vi "CRYO_MASTER_FULL_RUN3.vi"() -> ()   [LabVIEW 2017] (continued)
            n626 = Index Array(array=w1254, index=w1253) -> (element=→"TIP7":dbl)
          }
          frame #44 {
            n627 = Search 1D Array(1D array=w1261, element=T14."TTH1" ("SensorLocations")) -> (index of element=w1258:i32)  [unwired: 1 in]
            n628 = Index Array(array=w1259, index=w1258) -> (element=→"TTH1":dbl)
          }
          frame #45 {
            n629 = Search 1D Array(1D array=w1266, element=T14."TTH2" ("SensorLocations")) -> (index of element=w1263:i32)  [unwired: 1 in]
            n630 = Index Array(array=w1264, index=w1263) -> (element=→"TTH2":dbl)
          }
          frame #46 {
            n631 = Search 1D Array(1D array=w1271, element=T14."TTH3" ("SensorLocations")) -> (index of element=w1268:i32)  [unwired: 1 in]
            n632 = Index Array(array=w1269, index=w1268) -> (element=→"TTH3":dbl)
          }
          frame #47 {
            n633 = Search 1D Array(1D array=w1276, element=T14."TTH4" ("SensorLocations")) -> (index of element=w1273:i32)  [unwired: 1 in]
            n634 = Index Array(array=w1274, index=w1273) -> (element=→"TTH4":dbl)
          }
          frame #48 {
            n635 = Search 1D Array(1D array=w1281, element="SensorLocation 1") -> (index of element=w1278:i32)  [unwired: 1 in]
            n636 = Index Array(array=w1279, index=w1278) -> (element=→"Temperature 1":dbl)
          }
          frame #49 {
            n637 = Search 1D Array(1D array=w1286, element="SensorLocation 2") -> (index of element=w1283:i32)  [unwired: 1 in]
            n638 = Index Array(array=w1284, index=w1283) -> (element=→"Temperature 2":dbl)
          }
        }
      }
      frame #1 {
        n639 = stacked-sequence {
          tunnel: w1288 -> [w1293 w1298 w1303 w1308 w1313 w1318 w1323 w1328 w1333 w1338 w1343 w1348 w1353 w1358 w1363 w1368 w1373 w1378 w1383]
          tunnel: w1287 -> [w1290 w1296 w1302 w1307 w1312 w1316 w1321 w1326 w1331 w1336 w1341 w1346 w1350 w1355 w1360 w1365 w1370 w1375 _]
          tunnel: w1287 -> [_ _ _ _ _ _ _ _ _ _ _ _ _ _ _ _ _ _ w1381]
          frame #0 {
            n640 = Search 1D Array(1D array=w1293, element="Insulation vacuum") -> (index of element=w1291:i32)  [unwired: 1 in]
            n641 = Index Array(array=w1290, index=w1291) -> (element=→"P_ins" →"P (insulation)":dbl)
          }
          frame #1 {
            n642 = Search 1D Array(1D array=w1298, element="4K reservoir pressure") -> (index of element=w1295:i32)  [unwired: 1 in]
            n643 = Index Array(array=w1296, index=w1295) -> (element=→"P_4Kres" →"P (4K reservoir)":dbl)
          }
          frame #2 {
            n644 = Search 1D Array(1D array=w1303, element="3He inlet pressure") -> (index of element=w1301:i32)  [unwired: 1 in]
            n645 = Index Array(array=w1302, index=w1301) -> (element=→"P_3HeIN" →"P (3He IN)":dbl)
          }
          frame #3 {
            n646 = Search 1D Array(1D array=w1308, element="Shield return press.") -> (index of element=w1306:i32)  [unwired: 1 in]
            n647 = Index Array(array=w1307, index=w1306) -> (element=→"P_SldRTN" →"P (shield return)":dbl)
          }
          frame #4 {
            n648 = Search 1D Array(1D array=w1313, element="3He pot pressure") -> (index of element=w1311:i32)  [unwired: 1 in]
            n649 = Index Array(array=w1312, index=w1311) -> (element=→"P_3Hepot" →"P (3He pot)":dbl)
          }
          frame #5 {
            n650 = Search 1D Array(1D array=w1318, element="1Kpot pressure") -> (index of element=w1315:i32)  [unwired: 1 in]
            n651 = Index Array(array=w1316, index=w1315) -> (element=→"P_1Kpot" →"P (1K pot)":dbl)
          }
          frame #6 {
            n652 = Search 1D Array(1D array=w1323, element="Dewar pressure") -> (index of element=w1320:i32)  [unwired: 1 in]
            n653 = Index Array(array=w1321, index=w1320) -> (element=→"P_Dewar" →"P (Dewar)":dbl)
          }
          frame #7 {
            n654 = Search 1D Array(1D array=w1328, element="HEX7 out pressure") -> (index of element=w1325:i32)  [unwired: 1 in]
            n655 = Index Array(array=w1326, index=w1325) -> (element=→"P_HEX7OUT" →"P (HEX7 out)":dbl)
          }
          frame #8 {
            n656 = Search 1D Array(1D array=w1333, element="Diff pressure HEX4") -> (index of element=w1330:i32)  [unwired: 1 in]
            n657 = Index Array(array=w1331, index=w1330) -> (element=→"DP_HEX4" →"DP HEX4":dbl)
          }
          frame #9 {
            n658 = Search 1D Array(1D array=w1338, element="Diff pressure HEX5") -> (index of element=w1335:i32)  [unwired: 1 in]
            n659 = Index Array(array=w1336, index=w1335) -> (element=→"DP_HEX5" →"DP HEX5":dbl)
          }
          frame #10 {
            n660 = Search 1D Array(1D array=w1343, element="3He pump exhaust flow") -> (index of element=w1340:i32)  [unwired: 1 in]
            n661 = Index Array(array=w1341, index=w1340) -> (element=→"F_1" →"F1 (3He pump exhaust) flow":dbl)
          }
          frame #11 {
            n662 = Search 1D Array(1D array=w1348, element="Shield flow") -> (index of element=w1345:i32)  [unwired: 1 in]
            n663 = Index Array(array=w1346, index=w1345) -> (element=→"F_2" →"F2 (shield flow)":dbl)
          }
          frame #12 {
            n664 = Search 1D Array(1D array=w1353, element="4He return flow from HEX7") -> (index of element=w1351:i32)  [unwired: 1 in]
            n665 = Index Array(array=w1350, index=w1351) -> (element=→"F_3" →"F3 (4He rtn flw via HEX7)":dbl)
          }
          frame #13 {
            n666 = Search 1D Array(1D array=w1358, element="3He incoming flow into HEX7") -> (index of element=w1356:i32)  [unwired: 1 in]
            n667 = Index Array(array=w1355, index=w1356) -> (element=→"F_4" →"F4 (3He in to HEX7)":dbl)
          }
          frame #14 {
            n668 = Search 1D Array(1D array=w1363, element="1Kpot pump exhaust flow") -> (index of element=w1361:i32)  [unwired: 1 in]
            n669 = Index Array(array=w1360, index=w1361) -> (element=→"F_5" →"F5 (1K pump ex.)":dbl)
          }
          frame #15 {
            n670 = Search 1D Array(1D array=w1368, element="4K reservoir level") -> (index of element=w1366:i32)  [unwired: 1 in]
            n671 = Index Array(array=w1365, index=w1366) -> (element=→"L3" →"He level (4K)":dbl)
          }
          frame #16 {
            n672 = Search 1D Array(1D array=w1373, element="1K pot level") -> (index of element=w1371:i32)  [unwired: 1 in]
            n673 = Index Array(array=w1370, index=w1371) -> (element=→"L(1K) (a1)" →"He level (1K)":dbl)
          }
          frame #17 {
            n674 = Search 1D Array(1D array=w1378, element="1K pot (b)") -> (index of element=w1376:i32)  [unwired: 1 in]
            n675 = Index Array(array=w1375, index=w1376) -> (element=→"1K pot(b1)" →"He level (1K) b":dbl)
          }
          frame #18 {
            n676 = case shown="False" TRUE {
              tunnel: w1383 -> [w1388 _]
              tunnel: "3He pot" -> [w1387 w1392]
              tunnel: w1381 -> [w1385 _]
              tunnel: [w1384 w1391] -> w1380
              frame False {
                n677 = Search 1D Array(1D array=w1388, element=w1387) -> (index of element=w1386:i32)  [unwired: 1 in]
                n678 = Index Array(array=w1385, index=w1386) -> (element=w1384:dbl)
              }
              frame True {
                n679 = local read "Labels (HP34401 LM)"() -> (w1393:string[])
                n680 = local read "LastData (HP34401 LM)"() -> (w1389:dbl[])
                n681 = Search 1D Array(1D array=w1393, element=w1392) -> (index of element=w1390:i32)  [unwired: 1 in]
                n682 = Index Array(array=w1389, index=w1390) -> (element=w1391:dbl)
              }
            }
            "3He pot level" <- w1380
            "He level (3He)" <- w1380
          }
        }
      }
    }
    n683 = case shown="True" w848 {
      tunnel: [w1954 w1966] -> w908
      tunnel: [w1944 w1965] -> w916
      tunnel: [w1953 w1964] -> w909
      tunnel: [w1952 timestamp[] [] ("TimeArray")] -> w878
      tunnel: [w1951 dbl[][] [] ("DataArray")] -> w876
      tunnel: w918 -> [w1950 w1961]
      tunnel: w917 -> [w1949 w1960]
      tunnel: w842 -> [w1945 _]
      tunnel: w845 -> [_ w1955]
      frame False {
        n684 = local read "Record interval"() -> (w1942:i64)
        n685 = call-dynamic "LSI336Data_measure.vi"("LSI336Data in"=w1950, "MeasurementIndex"=w1945, "error in (no error)"=w1949, "save every ... measurements"=w1942) -> ("Active?"=→"Active?\n(LSI336)":bool[], "TimeMeasuremeent"=→"Time of Last Measurement (LSI336)":timestamp, "LSI336Data out"=w1953:refnum<class "LSI336Data.lvclass">, "LastData"=→"Last Data \nLSI336":dbl[], "LastMeasurementConfig"=→"LastMeasurementConfig (336)":T17, "DataArray"=w1951:dbl[][], "Status"=w1944:u16, "TimeArray"=w1952:timestamp[], "error out"=w1954:errorcluster)  [unwired: 3 in]
      }
      frame True {
        n686 = local read "RUN Identifier"() -> (w1956:string)
        n687 = call-dynamic "LSI336Data_initialize.vi"("LSI336Data in"=w1961, "RunIdentifier"=w1956, "InstName"="InstName (LSI336)", "FileFormat"="FileFormat (336)", "LSI336Settings(X, Y)"="LSI336Settings(X,Y)", "error in (no error)"=w1960, "base path"=w1955) -> ("LSI336Data out"=w1964:refnum<class "LSI336Data.lvclass">, "Status"=w1965:T7, "AllLabels"=→"Labels LSI336":string[], "error out"=w1966:errorcluster)  [unwired: 5 in]
      }
    }
    "LSI336 Status" <- w916
    "error out (LSI336)" <- w908
    "TimeArray (LSI336)" <- w878
    "DataArray (336)" <- w876
    n688 = local read "Labels (HP34401 LM) 2"() -> (w841:string[])
    n689 = case shown="False" w848 {
      tunnel: [w2059 w2074] -> w921
      tunnel: [w2054 w2073] -> w938
      tunnel: [w2057 w2072] -> w922
      tunnel: w842 -> [w2058 _]
      tunnel: w937 -> [w2048 w2067]
      tunnel: w936 -> [w2049 w2066]
      tunnel: w845 -> [_ w2065]
      tunnel: [w2046 timestamp[] [] ("TimeArray")] -> w935
      tunnel: [w2045 dbl[][] [] ("DataArray")] -> w934
      frame False {
        w2052 = 24 ("index")
        n690 = local read "Record interval"() -> (w2043:i64)
        n691 = call-dynamic "LSI218Data_measure.vi"("LSI218Data in"=w2049, "MeasurementIndex"=w2058, "error in (no error)"=w2048, "save every ... measurements"=w2043) -> ("TimeMeasuremeent"=→"Time of Last Measurement (LSI218)":timestamp, "Active?"=w2053:bool[], "LSI218Data out"=w2057:refnum<class "LSI218Data.lvclass">, "LastMeasurementConfig"=→"LastMeasurementConfig (218)":T17, "LastData"=w2047:dbl[], "Status"=w2054:u16, "TimeArray"=w2046:timestamp[], "DataArray"=w2045:dbl[][], "error out"=w2059:errorcluster)  [unwired: 3 in]
        "LastData (LSI218)" <- w2047
        n692 = Split 1D Array(array=w2053, index=w2052) -> (first subarray=→"Active?\n (1)":bool[], second subarray=→"Active?\n(2)":bool[])
        n693 = Split 1D Array(array=w2047, index=w2052) -> (first subarray=→"Last Data \nLSI218 (1)":dbl[], second subarray=→"Last Data \nLSI218 (2)":dbl[])
      }
      frame True {
        n694 = local read "RUN Identifier"() -> (w2061:string)
        n695 = call-dynamic "LSI218Data_initialize.vi"("LSI218Settings(A-F)"="LSI218Settings(A-F)", "FileFormat"="FileFormat (218)", "base path"=w2065, "error in (no error)"=w2067, "InstName"="InstName (LSI218)", "RunIdentifier"=w2061, "LSI218Data in"=w2066) -> ("error out"=w2074:errorcluster, "Status"=w2073:T7, "AllLabels"=w2064:string[], "LSI218Data out"=w2072:refnum<class "LSI218Data.lvclass">)  [unwired: 1 in]
        n696 = Split 1D Array(array=w2064, index=24) -> (first subarray=→"Labels LSI218 (1)":string[], second subarray=→"Labels LSI218 (2)":string[])
      }
    }
    "LSI218 Status" <- w938
    "error out (LSI218)" <- w921
    n697 = case shown="True" w848 {
      tunnel: w847 -> [w1010 w1024]
      tunnel: [w1007 w1023] -> w846
      tunnel: w845 -> [_ w1021]
      tunnel: w844 -> [w1009 w1020]
      tunnel: [w1006 w1017] -> w843
      tunnel: w842 -> [w1008 _]
      tunnel: [w1004 dbl[][] [] ("LastDataArray")] -> w839
      tunnel: [w1003 timestamp[] [] ("LastTimeArray")] -> w837
      frame False {
        n698 = call-dynamic "LMData_measure.vi"("error in (no error)"=w1009, "MeasurementInterval(>0)"="LM measurement interval (>0)", "MeasurementIndex"=w1008, "LMData in"=w1010) -> ("error out"=w1006:errorcluster, "LastDataArray"=w1004:dbl[][], "LastMeasurement"=→"LastData (HP34401 LM)":dbl[], "LMData out"=w1007:refnum<class "LMData.lvclass">, "LastTimeArray"=w1003:timestamp[])  [unwired: 3 in]
      }
      frame True {
        n699 = local read "RUN Identifier"() -> (w1022:string)
        n700 = call-dynamic "LMData_initialize.vi"("LMData in"=w1024, "VISA resource name"="VISA (HP34401 LM)", "Labels"="Labels (HP34401 LM)", "FileFormat"="FileFormat (HP34401 LM)", "RunIdentifier"=w1022, "InstName"="InstName (HP34401 LM)", "base path"=w1021, "error in (no error)"=w1020, "LevelCalibration (R0, R1, L0, L1)"="LevelCalibration (R0, R1, L0, L1)", "Active?"="Active? (HP34401 LM)") -> ("LMData out"=w1023:refnum<class "LMData.lvclass">, "error out"=w1017:errorcluster)  [unwired: 4 in]
        "Labels (HP34401 LM) 2" <- "Labels (HP34401 LM)"
      }
    }
    "error out (HP34401 LM)" <- w843
    n701 = Array Size(array=w841) -> (size(s)=w840:i32)
    n702 = for {
      N: w840 -> [_]
      tunnel: w839 -> [w964]
      shift-right: [w951] -> w833
      shift-left: w838 -> [w950]
      shift-right: [w954] -> w835
      shift-left: w838 -> [w955]
      shift-right: [w958] -> w836
      shift-left: w838 -> [w959]
      shift-right: [w953] -> w834
      shift-left: w838 -> [w952]
      tunnel: w837 -> [w962]
      i -> [w963]
      n703 = local read "Plot selecter (HP34401A)\n    1      2     3     4"() -> (w969:bool[][])
      n704 = Index Array(array=w964, index (col)=w963) -> (element=w961:dbl[])  [unwired: 1 in]
      n705 = Bundle("LastTimeArray"=w962, "LastDataArray"=w961) -> (w960:T29)  [unwired: 1 in]
      n706 = Index Array(array=w969, index (row) #1=w963, index (col) #1=0 ("disabled index (col)"), index (row) #2=w963, index (col) #2=1 ("index (col)"), index (row) #3=w963, index (col) #3=2 ("index (col)"), index (row) #4=w963, index (col) #4=3 ("disabled index (col)")) -> (element #1=w957:bool, element #2=w956:bool, element #3=w949:bool, element #4=w948:bool)
      n707 = stacked-sequence {
        tunnel: w960 -> [w971 w978 w989 w997]
        tunnel: w959 -> [w973 _ _ _]
        tunnel: [w972 _ _ _] -> w958
        tunnel: w957 -> [w970 _ _ _]
        tunnel: w956 -> [_ w981 _ _]
        tunnel: w955 -> [_ w980 _ _]
        tunnel: [_ w979 _ _] -> w954
        tunnel: [_ _ w988 _] -> w953
        tunnel: w952 -> [_ _ w987 _]
        tunnel: [_ _ _ w996] -> w951
        tunnel: w950 -> [_ _ _ w995]
        tunnel: w949 -> [_ _ w986 _]
        tunnel: w948 -> [_ _ _ w994]
        frame #0 {
          n708 = case shown="True" w970 {
            tunnel: w973 -> [w974 w977]
            tunnel: [w974 w976] -> w972
            tunnel: w971 -> [_ w975]
            frame False {
            }
            frame True {
              n709 = Build Array (concatenate)(w977, w975) -> (w976:T30)
            }
          }
        }
        frame #1 {
          n710 = case shown="True" w981 {
            tunnel: [w982 w985] -> w979
            tunnel: w980 -> [w982 w984]
            tunnel: w978 -> [_ w983]
            frame False {
            }
            frame True {
              n711 = Build Array (concatenate)(w984, w983) -> (w985:T30)
            }
          }
        }
        frame #2 {
          n712 = case shown="True" w986 {
            tunnel: [w990 w993] -> w988
            tunnel: w989 -> [_ w992]
            tunnel: w987 -> [w990 w991]
            frame False {
            }
            frame True {
              n713 = Build Array (concatenate)(w991, w992) -> (w993:T30)
            }
          }
        }
        frame #3 {
          n714 = case shown="True" w994 {
            tunnel: [w998 w1001] -> w996
            tunnel: w997 -> [_ w1000]
            tunnel: w995 -> [w998 w999]
            frame False {
            }
            frame True {
              n715 = Build Array (concatenate)(w999, w1000) -> (w1001:T30)
            }
          }
        }
      }
    }
    n716 = local read "Last Data \n(USB6210)"() -> (w862:dbl[])
    n717 = local read "Last Data \n(USB6218)"() -> (w863:dbl[])
    n718 = local read "All Labels (USB6210)"() -> (w865:string[])
    n719 = local read "All Labels (USB6218)"() -> (w864:string[])
    n720 = flat-sequence {
      tunnel: w892 -> [w1452]
      tunnel: [w1447] -> w891
      tunnel: [w1445] -> w890
      tunnel: [w1444] -> w889
      tunnel: [w1443] -> w888
      tunnel: w893 -> [w1439]
      frame #0 {
        w1446 = T25 [] ("appended array")
        n721 = Unbundle By Name(w1439) -> ("TimeArray"=w1435:timestamp[], "DataArrayConv"=w1450:dbl[][], "LDArray"=w1449:dbl[])
        "TimeArray (USB6218)" <- w1435
        n722 = Unbundle By Name(w1452) -> ("ReadLeakDet?"=w1451:bool, "LabelLD"=w1454:string, "Labels"=w1448:string[])  [unwired: 1 out]
        n723 = case shown="True" w1451 {
          tunnel: w1454 -> [_ w1462]
          tunnel: w1450 -> [w1456 w1461]
          tunnel: w1449 -> [_ w1460]
          tunnel: [w1456 w1459] -> w1437
          tunnel: w1448 -> [w1455 w1458]
          tunnel: [w1455 w1457] -> w1440
          frame False {
          }
          frame True {
            n724 = Build Array (concatenate)(w1461, w1460) -> (w1459:dbl[][])
            n725 = Build Array (concatenate)(w1458, w1462) -> (w1457:string[])
          }
        }
        "All Labels (USB6218)" <- w1440
        "DataArrayConv (USB6218)" <- w1437
        n726 = Array Size(array=w1435) -> (size(s)=→"TimeArray size (6218)":i32)
        n727 = local read "Plot selecter (USB6218)\n    1      2     3     4"() -> (w1442:bool[][])
        n728 = control-ref of="Plot selecter (USB6218)\n    1      2     3     4"() -> (w1438:refnum<vi>)
        n729 = Array Size(array=w1440) -> (size(s)=w1441:i32)
        n730 = Array Size(array=w1440) -> (size(s)=w1453:i32)
        n731 = Array Size(array=w1437) -> (size(s)=→"DataArraySize (6218)":i32[])
        n732 = property on="Property Node" class="Arr (strict)"(reference=w1438, "Number of Rows"=w1441) -> ()  [unwired: 1 in, 2 out]
        n733 = for {
          N: w1453 -> [_]
          tunnel: w1437 -> [w1483]
          tunnel: w1435 -> [w1484]
          shift-right: [w1478] -> w1445
          shift-left: w1446 -> [w1481]
          shift-right: [w1476] -> w1443
          shift-left: w1446 -> [w1479]
          shift-right: [w1477] -> w1447
          shift-left: w1446 -> [w1475]
          shift-right: [w1474] -> w1444
          shift-left: w1446 -> [w1473]
          tunnel: w1442 -> [w1472]
          i -> [w1467]
          n734 = Index Array(array=w1483, index (col)=w1467) -> (element=w1482:dbl[])  [unwired: 1 in]
          n735 = Index Array(array=w1472, index (row) #1=w1467, index (col) #1=0 ("index (row)"), index (row) #2=w1467, index (col) #2=1 ("index (row)"), index (row) #3=w1467, index (col) #3=2 ("index (row)"), index (row) #4=w1467, index (col) #4=3 ("index (row)")) -> (element #1=w1466:bool, element #2=w1465:bool, element #3=w1464:bool, element #4=w1463:bool)
          n736 = Bundle("TimeArray"=w1484, "DataArrayConv"=w1482) -> (w1480:T31)  [unwired: 1 in]
          n737 = stacked-sequence {
            tunnel: w1466 -> [w1488 _ _ _]
            tunnel: w1481 -> [_ w1496 _ _]
            tunnel: w1464 -> [_ _ w1504 _]
            tunnel: w1480 -> [w1485 w1494 w1503 w1509]
            tunnel: w1463 -> [_ _ _ w1512]
            tunnel: w1479 -> [_ _ _ w1511]
            tunnel: [_ _ _ w1510] -> w1476
            tunnel: [_ w1495 _ _] -> w1478
            tunnel: [w1487 _ _ _] -> w1477
            tunnel: w1475 -> [w1486 _ _ _]
            tunnel: [_ _ w1502 _] -> w1474
            tunnel: w1473 -> [_ _ w1501 _]
            tunnel: w1465 -> [_ w1493 _ _]
            frame #0 {
              n738 = case shown="True" w1488 {
                tunnel: [w1489 w1492] -> w1487
                tunnel: w1485 -> [_ w1491]
                tunnel: w1486 -> [w1489 w1490]
                frame False {
                }
                frame True {
                  n739 = Build Array (concatenate)(w1490, w1491) -> (w1492:T25)
                }
              }
            }
            frame #1 {
              n740 = case shown="True" w1493 {
                tunnel: w1496 -> [w1497 w1500]
                tunnel: [w1497 w1499] -> w1495
                tunnel: w1494 -> [_ w1498]
                frame False {
                }
                frame True {
                  n741 = Build Array (concatenate)(w1500, w1498) -> (w1499:T25)
                }
              }
            }
            frame #2 {
              n742 = case shown="True" w1504 {
                tunnel: [w1505 w1508] -> w1502
                tunnel: w1503 -> [_ w1507]
                tunnel: w1501 -> [w1505 w1506]
                frame False {
                }
                frame True {
                  n743 = Build Array (concatenate)(w1506, w1507) -> (w1508:T25)
                }
              }
            }
            frame #3 {
              n744 = case shown="True" w1512 {
                tunnel: [w1513 w1516] -> w1510
                tunnel: w1509 -> [_ w1515]
                tunnel: w1511 -> [w1513 w1514]
                frame False {
                }
                frame True {
                  n745 = Build Array (concatenate)(w1514, w1515) -> (w1516:T25)
                }
              }
            }
          }
        }
      }
    }
    n746 = case shown="True" "Digital Out ON?" {
      tunnel: w848 -> [_ w1655]
      tunnel: w898 -> [w1649 w1654]
      tunnel: [w1649 w1653] -> w897
      tunnel: w896 -> [_ w1652]
      tunnel: w845 -> [_ w1651]
      tunnel: w879 -> [_ w1650]
      frame False {
      }
      frame True {
        n747 = case shown="True" w1655 {
          tunnel: w1654 -> [w1673 w1856]
          tunnel: [w1673 w1869] -> w1653
          tunnel: w1652 -> [w1674 _]
          tunnel: w1651 -> [_ w1848]
          tunnel: w1650 -> [_ _]
          frame False {
            n748 = flat-sequence {
              frame #0 {
              }
            }
            n749 = case shown="\"USB6218AI\"" "AutoFill Source (P)" {
              tunnel: [w1677 w1678] -> w1659
              frame "USB6210", Default {
                n750 = local read "All Labels (USB6210)"() -> (w1677:string[])
              }
              frame "USB6218AI" {
                n751 = local read "All Labels (USB6218)"() -> (w1678:string[])
              }
            }
            n752 = case shown="\"USB6210\", Default" "AutoFill Source (L)" {
              tunnel: [w1675 w1676] -> w1656
              frame "USB6210", Default {
                n753 = local read "All Labels (USB6210)"() -> (w1675:string[])
              }
              frame "USB6218AI" {
                n754 = local read "All Labels (USB6218)"() -> (w1676:string[])
              }
            }
            n755 = Multiply(x="N for sampling", y=i64 2) -> (x*y=w1668:i64)
            n756 = local read "Cycle #"() -> (w1672:u32)
            n757 = Search 1D Array(1D array=w1659, element="Auto Fll Dewar P. label") -> (index of element=→"Target Index (P)":i32)  [unwired: 1 in]
            n758 = Search 1D Array(1D array=w1656, element="Auto Fll He L. label") -> (index of element=→"Target Index (L)":i32)  [unwired: 1 in]
            n759 = Add(x=w1668, y="Mov. Avg Interval") -> (x+y=w1670:i64)
            n760 = Greater?(x=w1672, y=w1670) -> (0:w1666:bool)
            n761 = And(x=w1666, y="Auto Fill ON?") -> (x .and. y?=w1664:bool)
            n762 = case shown="True" w1664 {
              tunnel: w1674 -> [_ w1712]
              tunnel: "Mov. Avg Interval" -> [_ w1698]
              tunnel: w1668 -> [_ w1685]
              tunnel: "N for sampling" -> [_ w1696]
              frame False {
              }
              frame True {
                n763 = local read "AutoFill Source (L)"() -> (w1679:T8)
                n764 = local read "AutoFill Source (P)"() -> (w1680:T8)
                n765 = case shown="\"USB6218AI\"" w1680 {
                  tunnel: [w1716 w1717] -> w1681
                  frame "USB6210", Default {
                    n766 = local read "DataArrayConv (USB6210)"() -> (w1716:dbl[][])
                  }
                  frame "USB6218AI" {
                    n767 = local read "DataArrayConv (USB6218)"() -> (w1717:dbl[][])
                  }
                }
                n768 = case shown="\"USB6210\", Default" w1679 {
                  tunnel: [w1714 w1715] -> w1683
                  frame "USB6210", Default {
                    n769 = local read "DataArrayConv (USB6210)"() -> (w1714:dbl[][])
                  }
                  frame "USB6218AI" {
                    n770 = local read "DataArrayConv (USB6218)"() -> (w1715:dbl[][])
                  }
                }
                n771 = local read "Pstd"() -> (→"Pstd history":dbl)
                n772 = local read "Lstd"() -> (→"Lstd history":dbl)
                n773 = local read "Target Index (L)"() -> (w1684:i32)
                n774 = local read "Pav (Pa)"() -> (→"Pav history":dbl)
                n775 = local read "Lav (%)"() -> (→"Lav history":dbl)
                n776 = Index Array(array=w1683, index (col)=w1684) -> (element=w1682:dbl[])  [unwired: 1 in]
                n777 = local read "Target Index (P)"() -> (w1713:i32)
                n778 = Unbundle By Name(w1712) -> ("TimeArray"=w1711:timestamp[])
                n779 = Index Array(array=w1681, index (col)=w1713) -> (element=w1700:dbl[])  [unwired: 1 in]
                n780 = Delete From Array(array=w1700, length=w1685) -> (deleted portion=w1708:dbl[])  [unwired: 1 in, 1 out]
                n781 = Delete From Array(array=w1682, length=w1685) -> (deleted portion=w1695:dbl[])  [unwired: 1 in, 1 out]
                n782 = call "MovingAverage.vi"("Moving Average interval"=w1698, "Input Array"=w1682) -> ("M.A. Array"=w1697:dbl[])  [unwired: 9 in]
                n783 = call "MovingAverage.vi"("Moving Average interval"=w1698, "Input Array"=w1700) -> ("M.A. Array"=w1699:dbl[])  [unwired: 9 in]
                n784 = Delete From Array(array=w1699, length=w1685) -> (deleted portion=w1709:dbl[])  [unwired: 1 in, 1 out]
                n785 = Delete From Array(array=w1699, length=w1685) -> (deleted portion=w1705:dbl[])  [unwired: 1 in, 1 out]
                "Last N M.A. Pressures" <- w1705
                n786 = Delete From Array(array=w1697, length=w1685) -> (deleted portion=w1690:dbl[])  [unwired: 1 in, 1 out]
                "Last N M.A. Levels" <- w1690
                n787 = Delete From Array(array=w1711, length=w1685) -> (deleted portion=w1692:timestamp[])  [unwired: 1 in, 1 out]
                n788 = Bundle("TimeArray"=w1692, "DataArrayConv (USB6218)"=w1708) -> (w1707:T32)  [unwired: 1 in]
                n789 = Bundle("TimeArray"=w1692, "M.A. Array"=w1709) -> (w1710:T33)  [unwired: 1 in]
                n790 = Bundle("TimeArray"=w1692, "DataArrayConv (USB6218)"=w1695) -> (w1694:T32)  [unwired: 1 in]
                n791 = Bundle("TimeArray"=w1692, "M.A. Array"=w1690) -> (w1691:T33)  [unwired: 1 in]
                n792 = Array Size(array=w1705) -> (size(s)=w1704:i32)
                n793 = Greater Or Equal?(x=w1704, y=w1696) -> (x >= y?=w1703:bool)
                n794 = Build Array(w1707, w1710) -> (→"Dewar Pressure":T34)
                n795 = Build Array(w1694, w1691) -> (→"He Level":T34)
                n796 = case shown="True" w1703 {
                  tunnel: [w1821 w1826] -> w1689
                  tunnel: w1705 -> [_ w1827]
                  tunnel: w1690 -> [_ w1824]
                  tunnel: [w1821 w1822] -> w1688
                  frame False {
                    w1821 = nan ("mean")
                  }
                  frame True {
                    n797 = call <vilib>:"Std Deviation and Variance.vi"("X"=w1827) -> ("mean"=w1826:dbl, "standard deviation"=w1825:dbl)  [unwired: 1 in, 1 out]
                    n798 = call <vilib>:"Std Deviation and Variance.vi"("X"=w1824) -> ("mean"=w1822:dbl, "standard deviation"=w1823:dbl)  [unwired: 1 in, 1 out]
                    n799 = local write "Pstd"(w1825) -> ()
                    n800 = local write "Lstd"(w1823) -> ()
                    n801 = local write "Pav (Pa)"(w1826) -> ()
                    n802 = local write "Lav (%)"(w1822) -> ()
                  }
                }
                n803 = flat-sequence {
                  tunnel: w1689 -> [w1718]
                  tunnel: w1688 -> [w1719]
                  frame #0 {
                    n804 = flat-sequence {
                      tunnel: w1719 -> [w1721]
                      tunnel: w1718 -> [w1720]
                      tunnel: w1718 -> [w1789]
                      frame #0 {
                        n805 = stacked-sequence {
                          tunnel: w1721 -> [w1728 w1732 _ _ _ _]
                          tunnel: w1720 -> [_ _ w1746 w1755 w1764 w1773]
                          frame #0 {
                            n806 = local read "L_low (%)"() -> (w1727:dbl)
                            n807 = local read "Fill state"() -> (w1725:bool)
                            n808 = Less?(x=w1728, y=w1727) -> (x < y?=w1724:bool)
                            n809 = Equal?(x=w1725, y=FALSE) -> (x = y?=w1723:bool)
                            n810 = And(x=w1724, y=w1723) -> (x .and. y?=w1722:bool)
                            n811 = case shown="False" w1722 {
                              frame False {
                              }
                              frame True {
                                w1730 = TRUE ("Value (Signaling)")
                                n812 = property on="Fill state" class="Bool (strict)"("Val(Sgnl)"=w1730) -> ()  [unwired: 2 in, 2 out]
                                n813 = Not(x=w1730) -> (.not. x?=w1729:bool)
                                n814 = property on="Fill (false)" class="Bool (strict)"("Val(Sgnl)"=w1729) -> ()  [unwired: 2 in, 2 out]
                              }
                            }
                          }
                          frame #1 {
                            n815 = local read "L_high (%)"() -> (w1733:dbl)
                            n816 = local read "Fill state"() -> (w1736:bool)
                            n817 = Greater?(x=w1732, y=w1733) -> (0:w1731:bool)
                            n818 = Equal?(x=w1736, y=TRUE) -> (x = y?=w1735:bool)
                            n819 = And(x=w1731, y=w1735) -> (x .and. y?=w1734:bool)
                            n820 = case shown="True" w1734 {
                              frame False {
                              }
                              frame True {
                                w1738 = FALSE ("Value (Signaling)")
                                n821 = property on="Fill state" class="Bool (strict)"("Val(Sgnl)"=w1738) -> ()  [unwired: 2 in, 2 out]
                                n822 = Not(x=w1738) -> (.not. x?=w1739:bool)
                                n823 = property on="Fill (false)" class="Bool (strict)"("Val(Sgnl)"=w1739) -> ()  [unwired: 2 in, 2 out]
                              }
                            }
                          }
                          frame #2 {
                            n824 = local read "P_1_low (Pa)"() -> (w1745:dbl)
                            n825 = property on="state 1" class="Bool (strict)"() -> ("Value"=w1743:bool)  [unwired: 2 in, 2 out]
                            n826 = Less?(x=w1746, y=w1745) -> (x < y?=w1742:bool)
                            n827 = Equal?(x=w1743, y=FALSE) -> (x = y?=w1741:bool)
                            n828 = And(x=w1741, y=w1742) -> (x .and. y?=w1740:bool)
                            n829 = case shown="True" w1740 {
                              frame False {
                              }
                              frame True {
                                w1748 = TRUE ("Value (Signaling)")
                                n830 = property on="state 1" class="Bool (strict)"("Val(Sgnl)"=w1748) -> ()  [unwired: 2 in, 2 out]
                                n831 = Not(x=w1748) -> (.not. x?=w1747:bool)
                                n832 = property on="state 1 (false)" class="Bool (strict)"("Val(Sgnl)"=w1747) -> ()  [unwired: 2 in, 2 out]
                              }
                            }
                          }
                          frame #3 {
                            n833 = local read "P_1_high (Pa)"() -> (w1754:dbl)
                            n834 = property on="state 1" class="Bool (strict)"() -> ("Value"=w1752:bool)  [unwired: 2 in, 2 out]
                            n835 = Greater?(x=w1755, y=w1754) -> (0:w1751:bool)
                            n836 = Equal?(x=w1752, y=TRUE) -> (x = y?=w1750:bool)
                            n837 = And(x=w1750, y=w1751) -> (x .and. y?=w1749:bool)
                            n838 = case shown="True" w1749 {
                              frame False {
                              }
                              frame True {
                                w1757 = FALSE ("Value (Signaling)")
                                n839 = property on="state 1" class="Bool (strict)"("Val(Sgnl)"=w1757) -> ()  [unwired: 2 in, 2 out]
                                n840 = Not(x=w1757) -> (.not. x?=w1756:bool)
                                n841 = property on="state 1 (false)" class="Bool (strict)"("Val(Sgnl)"=w1756) -> ()  [unwired: 2 in, 2 out]
                              }
                            }
                          }
                          frame #4 {
                            n842 = local read "P_2_low (Pa)"() -> (w1763:dbl)
                            n843 = property on="state 2" class="Bool (strict)"() -> ("Value"=w1758:bool)  [unwired: 2 in, 2 out]
                            n844 = Less?(x=w1764, y=w1763) -> (x < y?=w1761:bool)
                            n845 = Equal?(x=w1758, y=FALSE) -> (x = y?=w1760:bool)
                            n846 = And(x=w1760, y=w1761) -> (x .and. y?=w1759:bool)
                            n847 = case shown="True" w1759 {
                              frame False {
                              }
                              frame True {
                                w1765 = TRUE ("Value (Signaling)")
                                n848 = property on="state 2" class="Bool (strict)"("Val(Sgnl)"=w1765) -> ()  [unwired: 2 in, 2 out]
                                n849 = Not(x=w1765) -> (.not. x?=w1766:bool)
                                n850 = property on="state 2 (false)" class="Bool (strict)"("Val(Sgnl)"=w1766) -> ()  [unwired: 2 in, 2 out]
                              }
                            }
                          }
                          frame #5 {
                            n851 = local read "P_2_high (Pa)"() -> (w1772:dbl)
                            n852 = property on="state 2" class="Bool (strict)"() -> ("Value"=w1767:bool)  [unwired: 2 in, 2 out]
                            n853 = Greater?(x=w1773, y=w1772) -> (0:w1770:bool)
                            n854 = Equal?(x=w1767, y=TRUE) -> (x = y?=w1769:bool)
                            n855 = And(x=w1769, y=w1770) -> (x .and. y?=w1768:bool)
                            n856 = case shown="True" w1768 {
                              frame False {
                              }
                              frame True {
                                w1774 = FALSE ("Value (Signaling)")
                                n857 = property on="state 2" class="Bool (strict)"("Val(Sgnl)"=w1774) -> ()  [unwired: 2 in, 2 out]
                                n858 = Not(x=w1774) -> (.not. x?=w1775:bool)
                                n859 = property on="state 2 (false)" class="Bool (strict)"("Val(Sgnl)"=w1775) -> ()  [unwired: 2 in, 2 out]
                              }
                            }
                          }
                        }
                      }
                      frame #1 {
                        n860 = property on="Fill state" class="Bool (strict)"() -> ("Value"=w1776:bool)  [unwired: 2 in, 2 out]
                        n861 = case shown="True" w1776 {
                          frame False {
                            n862 = property on="V1 (N.O.)" class="Bool (strict)"("Val(Sgnl)"=TRUE ("V1 (N.O.)")) -> ()  [unwired: 2 in, 2 out]
                            n863 = property on="V2 (N.C.)" class="Bool (strict)"("Val(Sgnl)"=FALSE ("Value (Signaling)")) -> ()  [unwired: 2 in, 2 out]
                          }
                          frame True {
                            n864 = property on="state 1" class="Bool (strict)"() -> ("Value"=w1780:bool)  [unwired: 2 in, 2 out]
                            n865 = property on="state 2" class="Bool (strict)"() -> ("Value"=w1779:bool)  [unwired: 2 in, 2 out]
                            n866 = case shown="True" w1780 {
                              frame False {
                                n867 = property on="V1 (N.O.)" class="Bool (strict)"("Val(Sgnl)"=TRUE ("Value (Signaling)")) -> ()  [unwired: 2 in, 2 out]
                                n868 = local write "Status V1 CTRL"(enum16{"Pressurize", "Release"}."Release" ("Status V1 CTRL")) -> ()
                              }
                              frame True {
                                n869 = property on="V1 (N.O.)" class="Bool (strict)"("Val(Sgnl)"=FALSE ("V1 (N.O.)")) -> ()  [unwired: 2 in, 2 out]
                                n870 = local write "Status V1 CTRL"(enum16{"Pressurize", "Release"}."Pressurize" ("Status V1 CTRL")) -> ()
                              }
                            }
                            n871 = case shown="True" w1779 {
                              frame False {
                                n872 = property on="V2 (N.C.)" class="Bool (strict)"("Val(Sgnl)"=FALSE ("Value (Signaling)")) -> ()  [unwired: 2 in, 2 out]
                                n873 = local write "Status V2 CTRL"(enum16{"Pressurize", "Release"}."Release" ("Status V2 CTRL")) -> ()
                              }
                              frame True {
                                n874 = property on="V2 (N.C.)" class="Bool (strict)"("Val(Sgnl)"=TRUE ("Value (Signaling)")) -> ()  [unwired: 2 in, 2 out]
                                n875 = local write "Status V2 CTRL"(enum16{"Pressurize", "Release"}."Pressurize" ("Status V2 CTRL")) -> ()
                              }
                            }
                          }
                        }
                      }
                      frame #2 {
                        n876 = Greater?(x=w1789, y="P_safelimit_high (Pa)") -> (0:w1791:bool)
                        n877 = Less?(x=w1789, y="P_safelimit_low (Pa)") -> (x < y?=w1793:bool)
                        n878 = Or(x=w1791, y=w1793) -> (x .or. y?=w1794:bool)
                        n879 = case shown="False" w1794 {
                          frame False {
                          }
                          frame True {
                            w1795 = FALSE ("Value (Signaling)")
                            w1797 = FALSE ("Value (Signaling)")
                            n880 = property on="V2 (N.C.)" class="Bool (strict)"("Val(Sgnl)"=FALSE ("V1 (N.O.)")) -> ()  [unwired: 2 in, 2 out]
                            n881 = property on="state 1" class="Bool (strict)"("Val(Sgnl)"=w1795) -> ()  [unwired: 2 in, 2 out]
                            n882 = property on="V1 (N.O.)" class="Bool (strict)"("Val(Sgnl)"=TRUE ("V1 (N.O.)")) -> ()  [unwired: 2 in, 2 out]
                            n883 = property on="state 2" class="Bool (strict)"("Val(Sgnl)"=w1797) -> ()  [unwired: 2 in, 2 out]
                            n884 = Not(x=w1795) -> (.not. x?=w1796:bool)
                            n885 = Not(x=w1797) -> (.not. x?=w1798:bool)
                            n886 = property on="state 1 (false)" class="Bool (strict)"("Val(Sgnl)"=w1796) -> ()  [unwired: 2 in, 2 out]
                            n887 = property on="state 2 (false)" class="Bool (strict)"("Val(Sgnl)"=w1798) -> ()  [unwired: 2 in, 2 out]
                          }
                        }
                      }
                    }
                  }
                  frame #1 {
                    n888 = property on="V2 (N.C.)" class="Bool (strict)"() -> ("Value"=w1808:bool)  [unwired: 2 in, 2 out]
                    n889 = property on="V1 (N.O.)" class="Bool (strict)"() -> ("Value"=w1819:bool)  [unwired: 2 in, 2 out]
                    n890 = local read "P_1_high (Pa)"() -> (w1813:dbl)
                    n891 = local read "P_2_high (Pa)"() -> (w1811:dbl)
                    n892 = local read "P_1_low (Pa)"() -> (w1814:dbl)
                    n893 = local read "P_2_low (Pa)"() -> (w1812:dbl)
                    n894 = local read "L_high (%)"() -> (w1809:dbl)
                    n895 = local read "L_low (%)"() -> (w1810:dbl)
                    n896 = local read "Pav (Pa)"() -> (w1802:dbl)
                    n897 = local read "Lav (%)"() -> (w1801:dbl)
                    n898 = Boolean To (0,1)(Boolean=w1808) -> (0, 1=w1807:i16)
                    n899 = Boolean To (0,1)(Boolean=w1819) -> (0, 1=w1820:i16)
                    n900 = local read "File Refn DewarCTRL"() -> (w1815:refnum<file>)
                    n901 = local read "Cycle #"() -> (w1818:u32)
                    n902 = Build Array(w1802, w1801, w1814, w1813, w1812, w1811, w1810, w1809, w1820, w1807) -> (w1806:dbl[])
                    n903 = Get Date/Time In Seconds() -> (seconds since 1Jan1904=w1816:timestamp)
                    n904 = call "FileWrite.vi"("DataArray"=w1806, "Time Stamp"=w1816, "Error In"=errorcluster {"status"=FALSE, "code"=0, "source"=""}, "FileFormat"=string[] ["%4.5e", "%4.2f", "%4.4e", "%4.4e", "%4.4e", "%4.4e", "%4.4e", "%d", "%d"] ("Array"), "Index"=w1818, "refnum in"=w1815) -> ("Error Out"=→"Error Out (Dewar CTRL":errorcluster, "Byte Stream File Refnum"=w1805:refnum<file>)  [unwired: 4 in]
                    n905 = local write "File Refn DewarCTRL"(w1805) -> ()
                  }
                }
              }
            }
          }
          frame True {
            w1866 = "_"
            w1829 = FALSE ("auto cleanup")
            w1831 = 1 items=["one channel for each line", "one channel for all lines"] ("line grouping")
            n906 = flat-sequence {
              frame #0 {
                w1883 = FALSE ("V1 (N.O.)")
                n907 = local write "V1 (N.O.)"(TRUE ("V1 (N.O.)")) -> ()
                n908 = local write "V2 (N.C.)"(FALSE ("V1 (N.O.)")) -> ()
                n909 = local write "state 2"(w1883) -> ()
                n910 = local write "state 1"(w1883) -> ()
                n911 = local write "Fill state"(w1883) -> ()
                n912 = Not(x=w1883) -> (.not. x?=w1885:bool)
                n913 = Not(x=w1883) -> (.not. x?=w1884:bool)
                n914 = local write "state 1 (false)"(w1884) -> ()
                n915 = local write "state 2 (false)"(w1884) -> ()
                n916 = local write "Fill (false)"(w1885) -> ()
              }
            }
            n917 = Get Date/Time In Seconds() -> (seconds since 1Jan1904=w1880:timestamp)
            n918 = call "LV_UNIXTIME.vi"("current time"=w1880) -> ("date/time string"=w1861:string)  [unwired: 9 in, 1 out]
            n919 = local read "RUN Identifier"() -> (w1828:string)
            n920 = Concatenate Strings(w1861, "_DO" ("new task name")) -> (w1877:string)
            n921 = Concatenate Strings(w1828, w1866, w1861, w1866) -> (w1847:string)
            n922 = Concatenate Strings(w1847, "DEWAR.csv" ("string")) -> (w1846:string)
            n923 = Concatenate Strings(w1847, "USB_DOUT.csv" ("string")) -> (w1850:string)
            n924 = Build Path(base path=w1848, name or relative path=w1846) -> (appended path=w1845:path)
            n925 = Build Path(base path=w1848, name or relative path=w1850) -> (appended path=w1865:path)
            n926 = Open/Create/Replace File(file path (use dialog)=w1865, error in=w1856, operation (0:open)=T24."open or create") -> (refnum out=w1863:refnum<file>, error out=w1855:errorcluster)  [unwired: 3 in, 1 out]
            n927 = call "FileIntialize.vi"("Error In"=w1855, "Labels"="DOUT Labels", "refnum in"=w1863) -> ("Error Out"=w1842:errorcluster, "File Refnum"=→"File Refn USB DO":refnum<file>)  [unwired: 7 in]
            n928 = Open/Create/Replace File(file path (use dialog)=w1845, error in=w1842, operation (0:open)=T24."open or create") -> (refnum out=w1853:refnum<file>, error out=w1854:errorcluster)  [unwired: 3 in, 1 out]
            n929 = call "FileIntialize.vi"("Error In"=w1854, "Labels"=string[] ["P_av", "L_av", "P_1_low", "P_1_high", "P_2_low", "P_2_high", "L_low", "L_high", "V1(NO)", "V2(NC)"], "refnum in"=w1853) -> ("Error Out"=w1841:errorcluster, "File Refnum"=→"File Refn DewarCTRL":refnum<file>)  [unwired: 7 in]
            n930 = Index Array(array="DOUT Physical CH", index #1=0 ("index"), index #2=1 ("index"), index #3=2 ("index"), index #4=3 ("index")) -> (element #1=w1859:tag, element #2=w1837:tag, element #3=w1836:tag, element #4=w1830:tag)
            n931 = call <vilib>:"DAQmx Create Task.vi"("new task name"=w1877, "auto cleanup"=FALSE, "error in"=w1841) -> ("task out"=w1878:refnum<k21>, "error out"=w1879:errorcluster)  [unwired: 11 in]
            n932 = call-poly <vilib>:"DAQmx Create Virtual Channel.vi"("task in"=w1878, "lines"=w1859, "line grouping"=w1831, "error in"=w1879) -> ("task out"=w1881:refnum<k21>, "error out"=w1882:errorcluster)  [unwired: 10 in]
            n933 = call-poly <vilib>:"DAQmx Create Virtual Channel.vi"("task in"=w1881, "lines"=w1837, "line grouping"=w1831, "error in"=w1882) -> ("task out"=w1868:refnum<k21>, "error out"=w1867:errorcluster)  [unwired: 10 in]
            n934 = call-poly <vilib>:"DAQmx Create Virtual Channel.vi"("task in"=w1868, "lines"=w1836, "line grouping"=w1831, "error in"=w1867) -> ("task out"=w1835:refnum<k21>, "error out"=w1834:errorcluster)  [unwired: 10 in]
            n935 = call-poly <vilib>:"DAQmx Create Virtual Channel.vi"("task in"=w1835, "lines"=w1830, "line grouping"=w1831, "error in"=w1834) -> ("task out"=w1832:refnum<k21>, "error out"=w1833:errorcluster)  [unwired: 10 in]
            n936 = call <vilib>:"DAQmx Start Task.vi"("task/channels in"=w1832, "error in"=w1833) -> ("task out"=w1872:refnum<k21>, "error out"=w1870:errorcluster)  [unwired: 12 in]
            n937 = Build Array(w1829, w1829, w1829, w1829) -> (w1873:bool[])
            n938 = call <vilib>:"DAQmx Write (Digital 1D Bool NChan 1Samp 1Line).vi"("task/channels in"=w1872, "data"=w1873, "timeout"=10.0, "error in"=w1870) -> ("task out"=→"DOUT task out":refnum<k21>, "error out"=w1869:errorcluster)  [unwired: 9 in, 1 out]
          }
        }
      }
    }
    "error out (USB6210/6218 DOUT)" <- w897
    n939 = Build Array (concatenate)(w862, w863) -> (w860:dbl[])
    n940 = Build Array (concatenate)(w865, w864) -> (w861:string[])
    n941 = flat-sequence {
      tunnel: w944 -> [w1533]
      tunnel: [w1528] -> w932
      tunnel: [w1526] -> w930
      tunnel: [w1525] -> w927
      tunnel: [w1524] -> w925
      tunnel: w896 -> [w1519]
      frame #0 {
        w1527 = T25 [] ("appended array")
        n942 = Unbundle By Name(w1519) -> ("TimeArray"=w1536:timestamp[], "DataArrayConv"=w1531:dbl[][], "LDArray"=w1530:dbl[])
        n943 = Unbundle By Name(w1533) -> ("ReadLeakDet?"=w1532:bool, "LabelLD"=w1535:string, "Labels"=w1529:string[])  [unwired: 1 out]
        n944 = case shown="True" w1532 {
          tunnel: w1535 -> [_ w1544]
          tunnel: w1531 -> [w1538 w1543]
          tunnel: w1530 -> [_ w1542]
          tunnel: [w1538 w1541] -> w1518
          tunnel: w1529 -> [w1537 w1540]
          tunnel: [w1537 w1539] -> w1521
          frame False {
          }
          frame True {
            n945 = Build Array (concatenate)(w1543, w1542) -> (w1541:dbl[][])
            n946 = Build Array (concatenate)(w1540, w1544) -> (w1539:string[])
          }
        }
        "All Labels (USB6210)" <- w1521
        "DataArrayConv (USB6210)" <- w1518
        n947 = control-ref of="Plot selecter (USB6210)\n    1      2     3     4"() -> (w1520:refnum<vi>)
        n948 = local read "Plot selecter (USB6210)\n    1      2     3     4"() -> (w1523:bool[][])
        n949 = Array Size(array=w1521) -> (size(s)=w1534:i32)
        n950 = Array Size(array=w1521) -> (size(s)=w1522:i32)
        n951 = Array Size(array=w1518) -> (size(s)=→"Data Array sizes (6210)":i32[])
        n952 = property on="Property Node" class="Arr (strict)"(reference=w1520, "Number of Rows"=w1522) -> ()  [unwired: 1 in, 2 out]
        n953 = for {
          N: w1534 -> [_]
          tunnel: w1518 -> [w1565]
          tunnel: w1536 -> [w1566]
          shift-right: [w1561] -> w1526
          shift-left: w1527 -> [w1564]
          shift-right: [w1559] -> w1524
          shift-left: w1527 -> [w1562]
          shift-right: [w1560] -> w1528
          shift-left: w1527 -> [w1558]
          shift-right: [w1557] -> w1525
          shift-left: w1527 -> [w1556]
          tunnel: w1523 -> [w1555]
          i -> [w1550]
          n954 = Index Array(array=w1565, index (col)=w1550) -> (element=w1545:dbl[])  [unwired: 1 in]
          n955 = Index Array(array=w1555, index (row) #1=w1550, index (col) #1=0 ("index (row)"), index (row) #2=w1550, index (col) #2=1 ("index (row)"), index (row) #3=w1550, index (col) #3=2 ("index (row)"), index (row) #4=w1550, index (col) #4=3 ("index (row)")) -> (element #1=w1549:bool, element #2=w1548:bool, element #3=w1547:bool, element #4=w1546:bool)
          n956 = Bundle("TimeArray"=w1566, "DataArrayConv"=w1545) -> (w1563:T31)  [unwired: 1 in]
          n957 = stacked-sequence {
            tunnel: w1549 -> [w1570 _ _ _]
            tunnel: w1564 -> [_ w1578 _ _]
            tunnel: w1547 -> [_ _ w1586 _]
            tunnel: w1563 -> [w1567 w1576 w1585 w1591]
            tunnel: w1546 -> [_ _ _ w1594]
            tunnel: w1562 -> [_ _ _ w1593]
            tunnel: [_ _ _ w1592] -> w1559
            tunnel: [_ w1577 _ _] -> w1561
            tunnel: [w1569 _ _ _] -> w1560
            tunnel: w1558 -> [w1568 _ _ _]
            tunnel: [_ _ w1584 _] -> w1557
            tunnel: w1556 -> [_ _ w1583 _]
            tunnel: w1548 -> [_ w1575 _ _]
            frame #0 {
              n958 = case shown="True" w1570 {
                tunnel: [w1571 w1574] -> w1569
                tunnel: w1567 -> [_ w1573]
                tunnel: w1568 -> [w1571 w1572]
                frame False {
                }
                frame True {
                  n959 = Build Array (concatenate)(w1572, w1573) -> (w1574:T25)
                }
              }
            }
            frame #1 {
              n960 = case shown="True" w1575 {
                tunnel: w1578 -> [w1579 w1582]
                tunnel: [w1579 w1581] -> w1577
                tunnel: w1576 -> [_ w1580]
                frame False {
                }
                frame True {
                  n961 = Build Array (concatenate)(w1582, w1580) -> (w1581:T25)
                }
              }
            }
            frame #2 {
              n962 = case shown="True" w1586 {
                tunnel: [w1587 w1590] -> w1584
                tunnel: w1585 -> [_ w1589]
                tunnel: w1583 -> [w1587 w1588]
                frame False {
                }
                frame True {
                  n963 = Build Array (concatenate)(w1588, w1589) -> (w1590:T25)
                }
              }
            }
            frame #3 {
              n964 = case shown="True" w1594 {
                tunnel: [w1595 w1598] -> w1592
                tunnel: w1591 -> [_ w1597]
                tunnel: w1593 -> [w1595 w1596]
                frame False {
                }
                frame True {
                  n965 = Build Array (concatenate)(w1596, w1597) -> (w1598:T25)
                }
              }
            }
          }
        }
      }
    }
    n966 = local read "Plot selecter LSI218(2)\n    1      2     3     4"() -> (w919:bool[][])
    n967 = local read "Plot selecter LSI218(1)\n    1      2     3     4"() -> (w920:bool[][])
    n968 = for {
      N: 48 -> [_]
      tunnel: w935 -> [w1987]
      tunnel: w934 -> [w1984]
      tunnel: w920 -> [w1968]
      tunnel: w919 -> [w1969]
      shift-right: [w1985] -> w933
      shift-left: w931 -> [w1986]
      shift-right: [w1980] -> w928
      shift-left: w931 -> [w1981]
      shift-right: [w1979] -> w926
      shift-left: w931 -> [w1978]
      shift-right: [w1977] -> w924
      shift-left: w931 -> [w1976]
      i -> [w1974]
      n969 = Index Array(array=w1984, index (col)=w1974) -> (element=w1983:dbl[])  [unwired: 1 in]
      n970 = Less?(x=w1974, y=24) -> (x < y?=w1975:bool)
      n971 = case shown="True" w1975 {
        tunnel: [w1992 w2010] -> w1973
        tunnel: [w1991 w2009] -> w1972
        tunnel: [w1990 w2007] -> w1971
        tunnel: [w1989 w2006] -> w1970
        tunnel: w1968 -> [_ w2005]
        tunnel: w1969 -> [w1999 _]
        tunnel: w1974 -> [w1994 w2002]
        frame False {
          n972 = Subtract(x=w1994, y=24) -> (x-y=w1998:i32)
          n973 = Index Array(array=w1999, index (row) #1=w1998, index (col) #1=0 ("index (row)"), index (row) #2=w1998, index (col) #2=1 ("index (row)"), index (row) #3=w1998, index (col) #3=2 ("index (row)"), index (row) #4=w1998, index (col) #4=3 ("index (row)")) -> (element #1=w1992:bool, element #2=w1991:bool, element #3=w1990:bool, element #4=w1989:bool)
        }
        frame True {
          n974 = Index Array(array=w2005, index (row) #1=w2002, index (col) #1=0 ("index (row)"), index (row) #2=w2002, index (col) #2=1 ("index (row)"), index (row) #3=w2002, index (col) #3=2 ("index (row)"), index (row) #4=w2002, index (col) #4=3 ("index (row)")) -> (element #1=w2010:bool, element #2=w2009:bool, element #3=w2007:bool, element #4=w2006:bool)
        }
      }
      n975 = Bundle("TimeArray"=w1987, "DataArray"=w1983) -> (w1982:T35)  [unwired: 1 in]
      n976 = stacked-sequence {
        tunnel: w1986 -> [w2014 _ _ _]
        tunnel: [w2013 _ _ _] -> w1985
        tunnel: w1982 -> [w2012 w2022 w2030 w2038]
        tunnel: w1981 -> [_ w2021 _ _]
        tunnel: [_ w2020 _ _] -> w1980
        tunnel: [_ _ w2029 _] -> w1979
        tunnel: w1978 -> [_ _ w2028 _]
        tunnel: [_ _ _ w2037] -> w1977
        tunnel: w1976 -> [_ _ _ w2036]
        tunnel: w1973 -> [w2011 _ _ _]
        tunnel: w1972 -> [_ w2019 _ _]
        tunnel: w1971 -> [_ _ w2027 _]
        tunnel: w1970 -> [_ _ _ w2035]
        frame #0 {
          n977 = case shown="False" w2011 {
            tunnel: w2012 -> [_ w2016]
            tunnel: w2014 -> [w2015 w2018]
            tunnel: [w2015 w2017] -> w2013
            frame False {
            }
            frame True {
              n978 = Build Array (concatenate)(w2018, w2016) -> (w2017:T4)
            }
          }
        }
        frame #1 {
          n979 = case shown="True" w2019 {
            tunnel: [w2023 w2026] -> w2020
            tunnel: w2022 -> [_ w2025]
            tunnel: w2021 -> [w2023 w2024]
            frame False {
            }
            frame True {
              n980 = Build Array (concatenate)(w2024, w2025) -> (w2026:T4)
            }
          }
        }
        frame #2 {
          n981 = case shown="True" w2027 {
            tunnel: [w2031 w2034] -> w2029
            tunnel: w2030 -> [_ w2033]
            tunnel: w2028 -> [w2031 w2032]
            frame False {
            }
            frame True {
              n982 = Build Array (concatenate)(w2032, w2033) -> (w2034:T4)
            }
          }
        }
        frame #3 {
          n983 = case shown="True" w2035 {
            tunnel: [w2039 w2042] -> w2037
            tunnel: w2038 -> [_ w2041]
            tunnel: w2036 -> [w2039 w2040]